vi "Dresden R2R Sputter 03.02.2018 IY24.vi"() -> ()   [LabVIEW 2009] (continued)
                                n20261 = Wait Until Next ms Multiple(millisecond multiple=u32 1000) -> ()  [unwired: 1 out]
                                }
                                frame #1 {
                                }
                                }
                                }
                                }
                              }
                              frame #1 {
                              }
                            }
                          }
                        }
                      }
                      frame #1 {
                      }
                    }
                  }
                }
              }
              frame #1 {
              }
            }
          }
          frame #2 {
            # "ROUTINE CHECK"
            n20262 = local read "Semi"() -> (w24846:bool)
            n20263 = case shown="False" w24846 {
              frame #0 {
                n20264 = stacked-sequence {
                  frame #0 {
                    n20265 = local read "Semi"() -> (w24847:bool)
                    n20266 = case shown="False" w24847 {
                      frame #0 {
                        n20267 = stacked-sequence {
                          frame #0 {
                            n20268 = local read "Semi"() -> (w24848:bool)
                            n20269 = case shown="False" w24848 {
                              frame #0 {
                                n20270 = while {
                                i -> [w24857]
                                stop <- w24852 stop-if-true
                                n20271 = Greater?(x=w24857, y=400) -> (0:w24855:bool)
                                n20272 = case shown="True" w24855 {
                                frame #0 {
                                }
                                frame #1 {
                                n20273 = local write "Error Message"("Start up process was cancelled.\nPlease check Chamber \nvacuum connections." ("Error Message")) -> ()
                                n20274 = local write "Semi"(TRUE ("Semi")) -> ()
                                }
                                }
                                n20275 = local read "Ch3_pressure"() -> (w24849:dbl)
                                n20276 = Less?(x=w24849, y=0.01) -> (x < y?=w24850:bool)
                                n20277 = case shown="False" w24850 {
                                tunnel: [TRUE FALSE] -> w24854
                                frame #0 {
                                }
                                frame #1 {
                                n20278 = Wait Until Next ms Multiple(millisecond multiple=u32 500) -> ()  [unwired: 1 out]
                                }
                                }
                                n20279 = local read "Semi"() -> (w24853:bool)
                                n20280 = Or(x=w24854, y=w24853) -> (x .or. y?=w24852:bool)
                                }
                              }
                              frame #1 {
                              }
                            }
                          }
                          frame #1 {
                            n20281 = local read "Semi"() -> (w24863:bool)
                            n20282 = case shown="False" w24863 {
                              frame #0 {
                                n20283 = Wait Until Next ms Multiple(millisecond multiple=u32 1000) -> ()  [unwired: 1 out]
                              }
                              frame #1 {
                              }
                            }
                          }
                        }
                      }
                      frame #1 {
                      }
                    }
                  }
                  frame #1 {
                    n20284 = local read "Semi"() -> (w24865:bool)
                    n20285 = case shown="False" w24865 {
                      frame #0 {
                        n20286 = stacked-sequence {
                          frame #0 {
                            n20287 = local read "Semi"() -> (w24866:bool)
                            n20288 = case shown="False" w24866 {
                              frame #0 {
                                n20289 = while {
                                i -> [w24873]
                                stop <- w24867 stop-if-true
                                n20290 = Greater?(x=w24873, y=80) -> (0:w24871:bool)
                                n20291 = case shown="True" w24871 {
                                frame #0 {
                                }
                                frame #1 {
                                n20292 = local write "Semi"(TRUE ("Semi")) -> ()
                                n20293 = local write "Error Message"("Start up process  cancelled\nbecause  CC not opened.\nPlease check CH3-CC connections." ("Error Message")) -> ()
                                }
                                }
                                n20294 = local read "Ch3_Cc_on_off_di"() -> (w24870:bool)
                                n20295 = case shown="False" w24870 {
                                tunnel: [TRUE FALSE] -> w24869
                                frame #0 {
                                }
                                frame #1 {
                                n20296 = Wait Until Next ms Multiple(millisecond multiple=u32 200) -> ()  [unwired: 1 out]
                                n20297 = local write "Ch3_Cc_on_off_do"(TRUE ("Ch1_Tp_bv_do")) -> ()
                                }
                                }
                                n20298 = local read "Semi"() -> (w24868:bool)
                                n20299 = Or(x=w24869, y=w24868) -> (x .or. y?=w24867:bool)
                                }
                              }
                              frame #1 {
                              }
                            }
                          }
                          frame #1 {
                            n20300 = local read "Semi"() -> (w24880:bool)
                            n20301 = case shown="False" w24880 {
                              frame #0 {
                                n20302 = while {
                                i -> [w24884]
                                stop <- w24881 stop-if-true
                                n20303 = Greater Or Equal?(x=w24884, y=150) -> (x >= y?=w24882:bool)
                                n20304 = Wait (ms)(milliseconds to wait=u32 200) -> ()  [unwired: 1 out]
                                n20305 = local read "Semi"() -> (w24886:bool)
                                n20306 = Compound Arithmetic op=OR(w24882, w24886) -> (w24881:bool)
                                }
                              }
                              frame #1 {
                              }
                            }
                          }
                          frame #2 {
                            n20307 = local read "Semi"() -> (w24887:bool)
                            n20308 = case shown="False" w24887 {
                              frame #0 {
                                n20309 = local write "Ch3_PA32"(TRUE ("P1")) -> ()
                                n20310 = local write "Ch3_PV21"(TRUE ("P1")) -> ()
                                n20311 = Wait Until Next ms Multiple(millisecond multiple=u32 2000) -> ()  [unwired: 1 out]
                              }
                              frame #1 {
                              }
                            }
                          }
                        }
                      }
                      frame #1 {
                      }
                    }
                  }
                  frame #2 {
                    n20312 = local read "Semi"() -> (w24891:bool)
                    n20313 = case shown="False" w24891 {
                      frame #0 {
                        n20314 = stacked-sequence {
                          frame #0 {
                            n20315 = local read "Semi"() -> (w24892:bool)
                            n20316 = case shown="False" w24892 {
                              frame #0 {
                                n20317 = while {
                                i -> [w24899]
                                stop <- w24893 stop-if-true
                                n20318 = Greater?(x=w24899, y=80) -> (0:w24897:bool)
                                n20319 = case shown="True" w24897 {
                                frame #0 {
                                }
                                frame #1 {
                                n20320 = local write "Semi"(TRUE ("Semi")) -> ()
                                n20321 = local write "Error Message"("Start up process  cancelled\nbecause  Trns-GV-BP not opened.\nPlease check Trns-GV-BP\n connections." ("Error Message")) -> ()
                                }
                                }
                                n20322 = local read "Ch3_Trns_gv_bp_di"() -> (w24896:bool)
                                n20323 = case shown="True" w24896 {
                                tunnel: [FALSE TRUE] -> w24895
                                frame #0 {
                                n20324 = Wait Until Next ms Multiple(millisecond multiple=u32 200) -> ()  [unwired: 1 out]
                                n20325 = local write "Ch3_Trns_gv_bp_do"(FALSE ("Ch1_Tp_bv_do")) -> ()
                                }
                                frame #1 {
                                }
                                }
                                n20326 = local read "Semi"() -> (w24894:bool)
                                n20327 = Or(x=w24895, y=w24894) -> (x .or. y?=w24893:bool)
                                }
                              }
                              frame #1 {
                              }
                            }
                          }
                          frame #1 {
                            n20328 = local read "Semi"() -> (w24906:bool)
                            n20329 = case shown="False" w24906 {
                              frame #0 {
                                n20330 = local write "Ch3_PA33"(TRUE ("P1")) -> ()
                                n20331 = local write "Ch3_PV22"(TRUE ("P1")) -> ()
                                n20332 = Wait Until Next ms Multiple(millisecond multiple=u32 2000) -> ()  [unwired: 1 out]
                              }
                              frame #1 {
                              }
                            }
                          }
                        }
                      }
                      frame #1 {
                      }
                    }
                  }
                  frame #3 {
                    n20333 = local read "Semi"() -> (w24910:bool)
                    n20334 = case shown="False" w24910 {
                      frame #0 {
                        n20335 = stacked-sequence {
                          frame #0 {
                            n20336 = local read "Semi"() -> (w24911:bool)
                            n20337 = case shown="False" w24911 {
                              frame #0 {
                                n20338 = while {
                                i -> [w24918]
                                stop <- w24912 stop-if-true
                                n20339 = Greater?(x=w24918, y=80) -> (0:w24916:bool)
                                n20340 = case shown="True" w24916 {
                                frame #0 {
                                }
                                frame #1 {
                                n20341 = local write "Semi"(TRUE ("Semi")) -> ()
                                n20342 = local write "Error Message"("Start up process  cancelled\nbecause  Trns-GV-BP2 not opened.\nPlease check Trns-GV-BP2\n connections." ("Error Message")) -> ()
                                }
                                }
                                n20343 = local read "Ch3_Trns_gv_bp2_di"() -> (w24915:bool)
                                n20344 = case shown="True" w24915 {
                                tunnel: [FALSE TRUE] -> w24914
                                frame #0 {
                                n20345 = local write "Ch3_Trns_gv_bp2_do"(FALSE ("Ch1_Tp_bv_do")) -> ()
                                n20346 = Wait Until Next ms Multiple(millisecond multiple=u32 200) -> ()  [unwired: 1 out]
                                }
                                frame #1 {
                                }
                                }
                                n20347 = local read "Semi"() -> (w24913:bool)
                                n20348 = Or(x=w24914, y=w24913) -> (x .or. y?=w24912:bool)
                                }
                              }
                              frame #1 {
                              }
                            }
                          }
                          frame #1 {
                            n20349 = local read "Semi"() -> (w24925:bool)
                            n20350 = case shown="False" w24925 {
                              frame #0 {
                                n20351 = local write "Ch3_PA34"(TRUE ("P1")) -> ()
                                n20352 = local write "Ch3_PV23"(TRUE ("P1")) -> ()
                                n20353 = Wait Until Next ms Multiple(millisecond multiple=u32 2000) -> ()  [unwired: 1 out]
                              }
                              frame #1 {
                              }
                            }
                          }
                        }
                      }
                      frame #1 {
                      }
                    }
                  }
                  frame #4 {
                    n20354 = local read "Semi"() -> (w24929:bool)
                    n20355 = case shown="False" w24929 {
                      frame #0 {
                        n20356 = stacked-sequence {
                          frame #0 {
                            n20357 = local read "Semi"() -> (w24930:bool)
                            n20358 = case shown="False" w24930 {
                              frame #0 {
                                n20359 = while {
                                i -> [w24939]
                                stop <- w24934 stop-if-true
                                n20360 = local read "Target_time_ch3"() -> (w24933:dbl)
                                n20361 = Multiply(x=w24933, y=7200) -> (x*y=w24931:dbl)
                                n20362 = Greater?(x=w24939, y=w24931) -> (0:w24938:bool)
                                n20363 = case shown="True" w24938 {
                                frame #0 {
                                }
                                frame #1 {
                                n20364 = local write "Semi"(TRUE ("Semi")) -> ()
                                }
                                }
                                n20365 = local read "Semi"() -> (w24937:bool)
                                n20366 = case shown="False" w24937 {
                                tunnel: [TRUE w24944] -> w24936
                                frame #0 {
                                }
                                frame #1 {
                                n20367 = local read "Target Pressure_ch3"() -> (w24943:dbl)
                                n20368 = local read "Ch3_pressure"() -> (w24942:dbl)
                                n20369 = Less Or Equal?(x=w24943, y=w24942) -> (x <= y?=w24941:bool)
                                n20370 = case shown="True" w24941 {
                                tunnel: [TRUE FALSE] -> w24944
                                frame #0 {
                                }
                                frame #1 {
                                n20371 = Wait Until Next ms Multiple(millisecond multiple=u32 750) -> ()  [unwired: 1 out]
                                }
                                }
                                }
                                }
                                n20372 = local read "Semi"() -> (w24935:bool)
                                n20373 = Or(x=w24936, y=w24935) -> (x .or. y?=w24934:bool)
                                }
                              }
                              frame #1 {
                              }
                            }
                          }
                          frame #1 {
                            n20374 = local read "Semi"() -> (w24949:bool)
                            n20375 = case shown="False" w24949 {
                              frame #0 {
                                n20376 = Wait (ms)(milliseconds to wait=u32 1000) -> ()  [unwired: 1 out]
                              }
                              frame #1 {
                              }
                            }
                          }
                          frame #2 {
                            n20377 = local read "Semi"() -> (w24951:bool)
                            n20378 = case shown="False" w24951 {
                              frame #0 {
                                n20379 = local write "Ch3_PA35"(TRUE ("P1")) -> ()
                                n20380 = local write "Ch3_PV24"(TRUE ("P1")) -> ()
                                n20381 = Wait Until Next ms Multiple(millisecond multiple=u32 1000) -> ()  [unwired: 1 out]
                              }
                              frame #1 {
                              }
                            }
                          }
                        }
                      }
                      frame #1 {
                      }
                    }
                  }
                }
              }
              frame #1 {
              }
            }
          }
          frame #3 {
            # "ROUTINE CHECK"
            n20382 = local read "Semi"() -> (w24955:bool)
            n20383 = case shown="False" w24955 {
              frame #0 {
                n20384 = stacked-sequence {
                  frame #0 {
                    n20385 = local read "Semi"() -> (w24956:bool)
                    n20386 = case shown="False" w24956 {
                      frame #0 {
                        w24957 = TRUE ("Visible")
                        n20387 = local write "system_status"("Start up was completed." ("system_status")) -> ()
                        n20388 = property on="final_mes_tab" class="TabCtl (strict)"("Visible"=w24957) -> ()  [unwired: 2 in, 2 out]
                        n20389 = local write "Cnt_Do_Buzzer"(w24957) -> ()
                        n20390 = Wait (ms)(milliseconds to wait=u32 3000 ("millisecond multiple")) -> ()  [unwired: 1 out]
                      }
                      frame #1 {
                      }
                    }
                  }
                  frame #1 {
                    n20391 = local read "Semi"() -> (w24960:bool)
                    n20392 = case shown="False" w24960 {
                      frame #0 {
                        w24961 = FALSE ("Visible")
                        n20393 = local write "system_status"("" ("system_status")) -> ()
                        n20394 = local write "Cnt_Do_Buzzer"(w24961) -> ()
                        n20395 = Wait (ms)(milliseconds to wait=u32 3000 ("millisecond multiple")) -> ()  [unwired: 1 out]
                        n20396 = property on="final_mes_tab" class="TabCtl (strict)"("Visible"=w24961) -> ()  [unwired: 2 in, 2 out]
                        n20397 = local write "Start_up_ch3"(w24961) -> ()
                      }
                      frame #1 {
                      }
                    }
                  }
                  frame #2 {
                    n20398 = local read "Semi"() -> (w24964:bool)
                    n20399 = case shown="False" w24964 {
                      frame #0 {
                        n20400 = stacked-sequence {
                          frame #0 {
                            n20401 = local write "Pps_code_entry"("PF331=" ("system_status")) -> ()
                          }
                          frame #1 {
                            n20402 = Wait (ms)(milliseconds to wait=u32 500) -> ()  [unwired: 1 out]
                          }
                          frame #2 {
                            n20403 = local write "Ppsok"(TRUE ("Ppsok")) -> ()
                          }
                          frame #3 {
                            n20404 = Wait (ms)(milliseconds to wait=u32 1000) -> ()  [unwired: 1 out]
                          }
                        }
                      }
                      frame #1 {
                      }
                    }
                  }
                  frame #3 {
                    n20405 = local read "Semi"() -> (w24969:bool)
                    n20406 = case shown="False" w24969 {
                      frame #0 {
                        n20407 = stacked-sequence {
                          frame #0 {
                            n20408 = local write "Pps_code_entry"("PF227=" ("system_status")) -> ()
                          }
                          frame #1 {
                            n20409 = Wait (ms)(milliseconds to wait=u32 500) -> ()  [unwired: 1 out]
                          }
                          frame #2 {
                            n20410 = local write "Ppsok"(TRUE ("Ppsok")) -> ()
                          }
                          frame #3 {
                            n20411 = Wait (ms)(milliseconds to wait=u32 1000) -> ()  [unwired: 1 out]
                          }
                        }
                      }
                      frame #1 {
                      }
                    }
                  }
                  frame #4 {
                    n20412 = local read "Semi"() -> (w24974:bool)
                    n20413 = case shown="False" w24974 {
                      frame #0 {
                        n20414 = stacked-sequence {
                          frame #0 {
                            n20415 = local write "Pps_code_entry"("PF330=" ("system_status")) -> ()
                          }
                          frame #1 {
                            n20416 = Wait (ms)(milliseconds to wait=u32 500) -> ()  [unwired: 1 out]
                          }
                          frame #2 {
                            n20417 = local write "Ppsok"(TRUE ("Ppsok")) -> ()
                          }
                          frame #3 {
                            n20418 = Wait (ms)(milliseconds to wait=u32 1000) -> ()  [unwired: 1 out]
                          }
                        }
                      }
                      frame #1 {
                      }
                    }
                  }
                  frame #5 {
                    n20419 = local read "Semi"() -> (w24979:bool)
                    n20420 = case shown="False" w24979 {
                      frame #0 {
                        w24980 = TRUE ("P018")
                        n20421 = local write "Ch3_PA36"(w24980) -> ()
                        n20422 = local write "Ch3_PV25"(w24980) -> ()
                        n20423 = Wait (ms)(milliseconds to wait=u32 1000) -> ()  [unwired: 1 out]
                      }
                      frame #1 {
                      }
                    }
                  }
                }
              }
              frame #1 {
              }
            }
          }
        }
      }
    }
    n20424 = case shown="True" "Shutdown_ch3" {
      frame #0 {
      }
      frame #1 {
        n20425 = local read "Semi"() -> (w23251:bool)
        n20426 = case shown="False" w23251 {
          frame #0 {
            n20427 = stacked-sequence {
              frame #0 {
                n20428 = local read "Semi"() -> (w23252:bool)
                n20429 = case shown="False" w23252 {
                  frame #0 {
                    n20430 = stacked-sequence {
                      frame #0 {
                        w23255 = FALSE
                        n20431 = local write "final_process_messages"("Shut Down process was completed." ("final_process_messages")) -> ()
                        n20432 = local write "system_status"("Shutting Down the System" ("system_status")) -> ()
                        n20433 = local write "Clean_shutdown_ch3"(TRUE) -> ()
                        n20434 = Wait (ms)(milliseconds to wait=u32 1000) -> ()  [unwired: 1 out]
                        "Yes 3" <- w23255
                        "No 3" <- w23255
                        "Cancel 3" <- w23255
                        "Close 3" <- w23255
                      }
                      frame #1 {
                        n20435 = call <vilib>:"Three Button Dialog.vi"("Right Button Text (\"Cancel\")"="Cancel" ("Right Button Text (\"Cancel\")"), "Center Button Text (\"No\")"="No" ("Center Button Text (\"No\")"), "Left Button Text (\"Yes\")"="Yes" ("Left Button Text (\"Yes\")"), "message"=" VENT the CHAMBER  \nLOAD or UNLOAD the substrate ? ") -> ("Which Button?"=w23261:T40)  [unwired: 7 in]
                        n20436 = case shown="\"Window Close\"" w23261 {
                          frame #0 {
                            n20437 = local write "Yes 3"(TRUE ("Close")) -> ()
                          }
                          frame #1 {
                            n20438 = local write "Close 3"(TRUE ("Close")) -> ()
                          }
                          frame #2 {
                            n20439 = local write "Cancel 3"(TRUE ("No")) -> ()
                          }
                          frame #3 {
                            n20440 = local write "No 3"(TRUE ("No")) -> ()
                          }
                        }
                      }
                      frame #2 {
                        n20441 = local read "Semi"() -> (w23267:bool)
                        n20442 = case shown="False" w23267 {
                          frame #0 {
                            n20443 = stacked-sequence {
                              frame #0 {
                                n20444 = local write "Error Message"("" ("Error Message")) -> ()
                              }
                              frame #1 {
                                n20445 = Wait (ms)(milliseconds to wait=u32 500) -> ()  [unwired: 1 out]
                              }
                              frame #2 {
                                n20446 = local write "Ppsok"(TRUE ("Ppsok")) -> ()
                              }
                              frame #3 {
                                n20447 = Wait (ms)(milliseconds to wait=u32 500) -> ()  [unwired: 1 out]
                              }
                            }
                          }
                          frame #1 {
                          }
                        }
                      }
                    }
                  }
                  frame #1 {
                  }
                }
              }
              frame #1 {
                n20448 = local read "Semi"() -> (w23272:bool)
                n20449 = case shown="False" w23272 {
                  frame #0 {
                    n20450 = local read "Cancel 3"() -> (w23274:bool)
                    n20451 = local read "Close 3"() -> (w23275:bool)
                    n20452 = Not Or(1:w23274, 2:w23275) -> (0:w23273:bool)
                    n20453 = case shown="True" w23273 {
                      frame #0 {
                        n20454 = local read "Semi"() -> (w23276:bool)
                        n20455 = case shown="False" w23276 {
                          frame #0 {
                          }
                          frame #1 {
                            n20456 = local write "system_status"("Semi-automatic is active" ("system_status")) -> ()
                            n20457 = local write "Shutdown_ch3"(FALSE ("Shutdown_ch1")) -> ()
                          }
                        }
                      }
                      frame #1 {
                        n20458 = local read "Yes 3"() -> (w23281:bool)
                        n20459 = local read "No 3"() -> (w23280:bool)
                        n20460 = Or(x=w23281, y=w23280) -> (x .or. y?=w23279:bool)
                        n20461 = case shown="True" w23279 {
                          frame #0 {
                          }
                          frame #1 {
                            n20462 = stacked-sequence {
                              frame #0 {
                                # "CLOSE & ZERO ROUTINES"
                                n20463 = local read "Semi"() -> (w23282:bool)
                                n20464 = case shown="False" w23282 {
                                frame #0 {
                                n20465 = stacked-sequence {
                                frame #0 {
                                n20466 = local read "Semi"() -> (w23283:bool)
                                n20467 = case shown="False" w23283 {
                                frame #0 {
                                w23285 = TRUE ("Dc_auto_off")
                                n20468 = local write "Dc_auto_off"(w23285) -> ()
                                n20469 = local write "Ar_auto_set_zero_ch3"(w23285) -> ()
                                n20470 = local write "system_status"("Shut Down in Progress for Chamber 3" ("system_status")) -> ()
                                n20471 = local write "final_process_messages"("Shut Down Process was completed for  Chamber 3." ("final_process_messages")) -> ()
                                n20472 = local write "Ch3_Sov_Ar_do"(FALSE ("Dc_auto_off")) -> ()
                                }
                                frame #1 {
                                }
                                }
                                }
                                frame #1 {
                                n20473 = local read "Semi"() -> (w23288:bool)
                                n20474 = case shown="False" w23288 {
                                frame #0 {
                                n20475 = Wait (ms)(milliseconds to wait=u32 2500) -> ()  [unwired: 1 out]
                                }
                                frame #1 {
                                }
                                }
                                }
                                frame #2 {
                                n20476 = local read "Semi"() -> (w23290:bool)
                                n20477 = case shown="False" w23290 {
                                frame #0 {
                                n20478 = local write "Ch3_Sov_Ar_do"(FALSE ("Ch1_Sov_Ar_do")) -> ()
                                n20479 = Wait (ms)(milliseconds to wait=u32 2500) -> ()  [unwired: 1 out]
                                n20480 = local write "RF_auto_off"(TRUE ("RF_auto_off")) -> ()
                                }
                                frame #1 {
                                }
                                }
                                }
                                frame #3 {
                                n20481 = local read "Semi"() -> (w23294:bool)
                                n20482 = case shown="False" w23294 {
                                frame #0 {
                                n20483 = Wait (ms)(milliseconds to wait=u32 1000) -> ()  [unwired: 1 out]
                                }
                                frame #1 {
                                }
                                }
                                }
                                }
                                }
                                frame #1 {
                                }
                                }
                              }
                              frame #1 {
                                # "STOP TP"
                                n20484 = local read "Semi"() -> (w23296:bool)
                                n20485 = case shown="False" w23296 {
                                frame #0 {
                                n20486 = stacked-sequence {
                                frame #0 {
                                n20487 = local read "Semi"() -> (w23297:bool)
                                n20488 = case shown="False" w23297 {
                                frame #0 {
                                n20489 = stacked-sequence {
                                frame #0 {
                                n20490 = local read "Semi"() -> (w23298:bool)
                                n20491 = case shown="False" w23298 {
                                frame #0 {
                                n20492 = local write "Tp3_auto_stop"(TRUE ("Tp1_auto_start")) -> ()
                                }
                                frame #1 {
                                }
                                }
                                }
                                frame #1 {
                                n20493 = local read "Semi"() -> (w23300:bool)
                                n20494 = case shown="False" w23300 {
                                frame #0 {
                                n20495 = Wait (ms)(milliseconds to wait=u32 1000) -> ()  [unwired: 1 out]
                                }
                                frame #1 {
                                }
                                }
                                }
                                frame #2 {
                                n20496 = local read "Semi"() -> (w23302:bool)
                                n20497 = case shown="False" w23302 {
                                frame #0 {
                                n20498 = while {
                                i -> [w23308]
                                stop <- w23304 stop-if-true
                                n20499 = local read "Tp3_stopped"() -> (w23306:bool)
                                n20500 = Greater?(x=w23308, y=120) -> (0:w23307:bool)
                                n20501 = local read "Semi"() -> (w23305:bool)
                                n20502 = Compound Arithmetic op=OR(w23305, w23306, w23307) -> (w23304:bool)
                                n20503 = Wait (ms)(milliseconds to wait=u32 500) -> ()  [unwired: 1 out]
                                }
                                }
                                frame #1 {
                                }
                                }
                                }
                                frame #3 {
                                n20504 = local read "Semi"() -> (w23310:bool)
                                n20505 = case shown="False" w23310 {
                                frame #0 {
                                n20506 = local read "Tp3_stopped"() -> (w23311:bool)
                                n20507 = case shown="False" w23311 {
                                frame #0 {
                                n20508 = local write "Tp3_auto_stop"(TRUE ("Pc_bv1_auto_open")) -> ()
                                }
                                frame #1 {
                                }
                                }
                                }
                                frame #1 {
                                }
                                }
                                }
                                frame #4 {
                                n20509 = local read "Semi"() -> (w23313:bool)
                                n20510 = case shown="False" w23313 {
                                frame #0 {
                                n20511 = local read "Tp3_stopped"() -> (w23314:bool)
                                n20512 = case shown="False" w23314 {
                                frame #0 {
                                n20513 = Wait (ms)(milliseconds to wait=u32 1000) -> ()  [unwired: 1 out]
                                }
                                frame #1 {
                                }
                                }
                                }
                                frame #1 {
                                }
                                }
                                }
                                frame #5 {
                                n20514 = local read "Semi"() -> (w23316:bool)
                                n20515 = case shown="False" w23316 {
                                frame #0 {
                                n20516 = while {
                                i -> [w23322]
                                stop <- w23318 stop-if-true
                                n20517 = local read "Tp3_stopped"() -> (w23320:bool)
                                n20518 = Greater?(x=w23322, y=120) -> (0:w23321:bool)
                                n20519 = local read "Semi"() -> (w23319:bool)
                                n20520 = Compound Arithmetic op=OR(w23319, w23320, w23321) -> (w23318:bool)
                                n20521 = Wait (ms)(milliseconds to wait=u32 500) -> ()  [unwired: 1 out]
                                }
                                }
                                frame #1 {
                                }
                                }
                                }
                                frame #6 {
                                n20522 = local read "Semi"() -> (w23324:bool)
                                n20523 = case shown="False" w23324 {
                                frame #0 {
                                n20524 = local read "Tp3_stopped"() -> (w23325:bool)
                                n20525 = case shown="False" w23325 {
                                frame #0 {
                                n20526 = local write "Error Message"("Shut Down process  cancelled\nbecause  TP not stopped.\nPlease check TP3 connections." ("Error Message")) -> ()
                                n20527 = local write "Semi"(TRUE ("Semi")) -> ()
                                }
                                frame #1 {
                                }
                                }
                                }
                                frame #1 {
                                }
                                }
                                }
                                }
                                }
                                frame #1 {
                                }
                                }
                                }
                                frame #1 {
                                n20528 = local read "Semi"() -> (w23328:bool)
                                n20529 = case shown="False" w23328 {
                                frame #0 {
                                n20530 = local write "Ch3_Sd1"(TRUE ("Ch1_Sd0")) -> ()
                                n20531 = Wait (ms)(milliseconds to wait=u32 1000) -> ()  [unwired: 1 out]
                                }
                                frame #1 {
                                }
                                }
                                }
                                }
                                }
                                frame #1 {
                                }
                                }
                              }
                              frame #2 {
                                # "CLOSE CC"
                                n20532 = local read "Semi"() -> (w23331:bool)
                                n20533 = case shown="False" w23331 {
                                frame #0 {
                                n20534 = stacked-sequence {
                                frame #0 {
                                n20535 = local read "Semi"() -> (w23332:bool)
                                n20536 = case shown="False" w23332 {
                                frame #0 {
                                n20537 = while {
                                i -> [w23338]
                                stop <- w23333 stop-if-true
                                n20538 = Greater?(x=w23338, y=25) -> (0:w23337:bool)
                                n20539 = case shown="True" w23337 {
                                frame #0 {
                                }
                                frame #1 {
                                n20540 = local write "Error Message"("Shut Down Process  cancelled\nbecause  CC not closed.\nPlease check CH3-CC connections." ("Error Message")) -> ()
                                n20541 = local write "Semi"(TRUE ("Semi")) -> ()
                                }
                                }
                                n20542 = local read "Ch3_Cc_on_off_di"() -> (w23336:bool)
                                n20543 = case shown="True" w23336 {
                                tunnel: [TRUE FALSE] -> w23334
                                frame #0 {
                                }
                                frame #1 {
                                n20544 = local write "Ch3_Cc_on_off_do"(FALSE ("Ch1_Ch_cc_on_off_di")) -> ()
                                n20545 = Wait Until Next ms Multiple(millisecond multiple=u32 200) -> ()  [unwired: 1 out]
                                }
                                }
                                n20546 = local read "Semi"() -> (w23335:bool)
                                n20547 = Or(x=w23334, y=w23335) -> (x .or. y?=w23333:bool)
                                }
                                }
                                frame #1 {
                                }
                                }
                                }
                                frame #1 {
                                n20548 = local read "Semi"() -> (w23346:bool)
                                n20549 = case shown="False" w23346 {
                                frame #0 {
                                n20550 = local write "Ch3_Sd2"(TRUE ("Ch1_Sd1")) -> ()
                                n20551 = Wait (ms)(milliseconds to wait=u32 1000) -> ()  [unwired: 1 out]
                                }
                                frame #1 {
                                }
                                }
                                }
                                }
                                }
                                frame #1 {
                                }
                                }
                              }
                              frame #3 {
                                # "CLOSE BG-BV"
                                n20552 = local read "Semi"() -> (w23349:bool)
                                n20553 = case shown="False" w23349 {
                                frame #0 {
                                n20554 = stacked-sequence {
                                frame #0 {
                                n20555 = local read "Semi"() -> (w23350:bool)
                                n20556 = case shown="False" w23350 {
                                frame #0 {
                                n20557 = while {
                                i -> [w23356]
                                stop <- w23351 stop-if-true
                                n20558 = Greater?(x=w23356, y=25) -> (0:w23355:bool)
                                n20559 = case shown="True" w23355 {
                                frame #0 {
                                }
                                frame #1 {
                                n20560 = local write "Error Message"("Shut Down Process  cancelled\nbecause  BG-BV not closed.\nPlease check BG-BV3 connections." ("Error Message")) -> ()
                                n20561 = local write "Semi"(TRUE ("Semi")) -> ()
                                }
                                }
                                n20562 = local read "Ch3_Bg_bv_di"() -> (w23354:bool)
                                n20563 = case shown="True" w23354 {
                                tunnel: [TRUE FALSE] -> w23352
                                frame #0 {
                                }
                                frame #1 {
                                n20564 = Wait Until Next ms Multiple(millisecond multiple=u32 200) -> ()  [unwired: 1 out]
                                n20565 = local write "Ch3_Bg_bv_do"(FALSE ("Ch1_Ch_cc_on_off_di")) -> ()
                                }
                                }
                                n20566 = local read "Semi"() -> (w23353:bool)
                                n20567 = Or(x=w23352, y=w23353) -> (x .or. y?=w23351:bool)
                                }
                                }
                                frame #1 {
                                }
                                }
                                }